vi "calibAnalyzeImage.vi"(0 "Input cluster":T1, 11 "error in":errorcluster) -> (4 "Output cluster":T1, 6 "Image out":T5(plugin-control), 12 "bottom border":sgl, 13 "left border":sgl, 14 "right border":sgl, 15 "error out":errorcluster)   [LabVIEW 2020]
doc: "Analyze image with a neural network, filter results and return calculated distance"
uses:
  controls/StateMachineVariables.ctl
  <vilib>/vision/Avi.llb/IMAQ AVI2 Refnum.ctl
  <vilib>/userDefined/High Color/IMAQdx.ctl
  <vilib>/vision/Deep Learning.llb/IMAQ DL Model Refnum.ctl
  <vilib>/vision/Image Controls.llb/IMAQ Image.ctl
  <vilib>/vision/Deep Learning.llb/IMAQ DL Model Detect Objects Node Names.ctl
  <vilib>/vision/Deep Learning.llb/IMAQ DL Model Label.ctl
  <vilib>/vision/NI_Vision_Development_Module.lvlib
panel:
  in  "Minimum Score Threshold":sgl=0.3 min=0 max=1 step=0.1 format="%.3g"
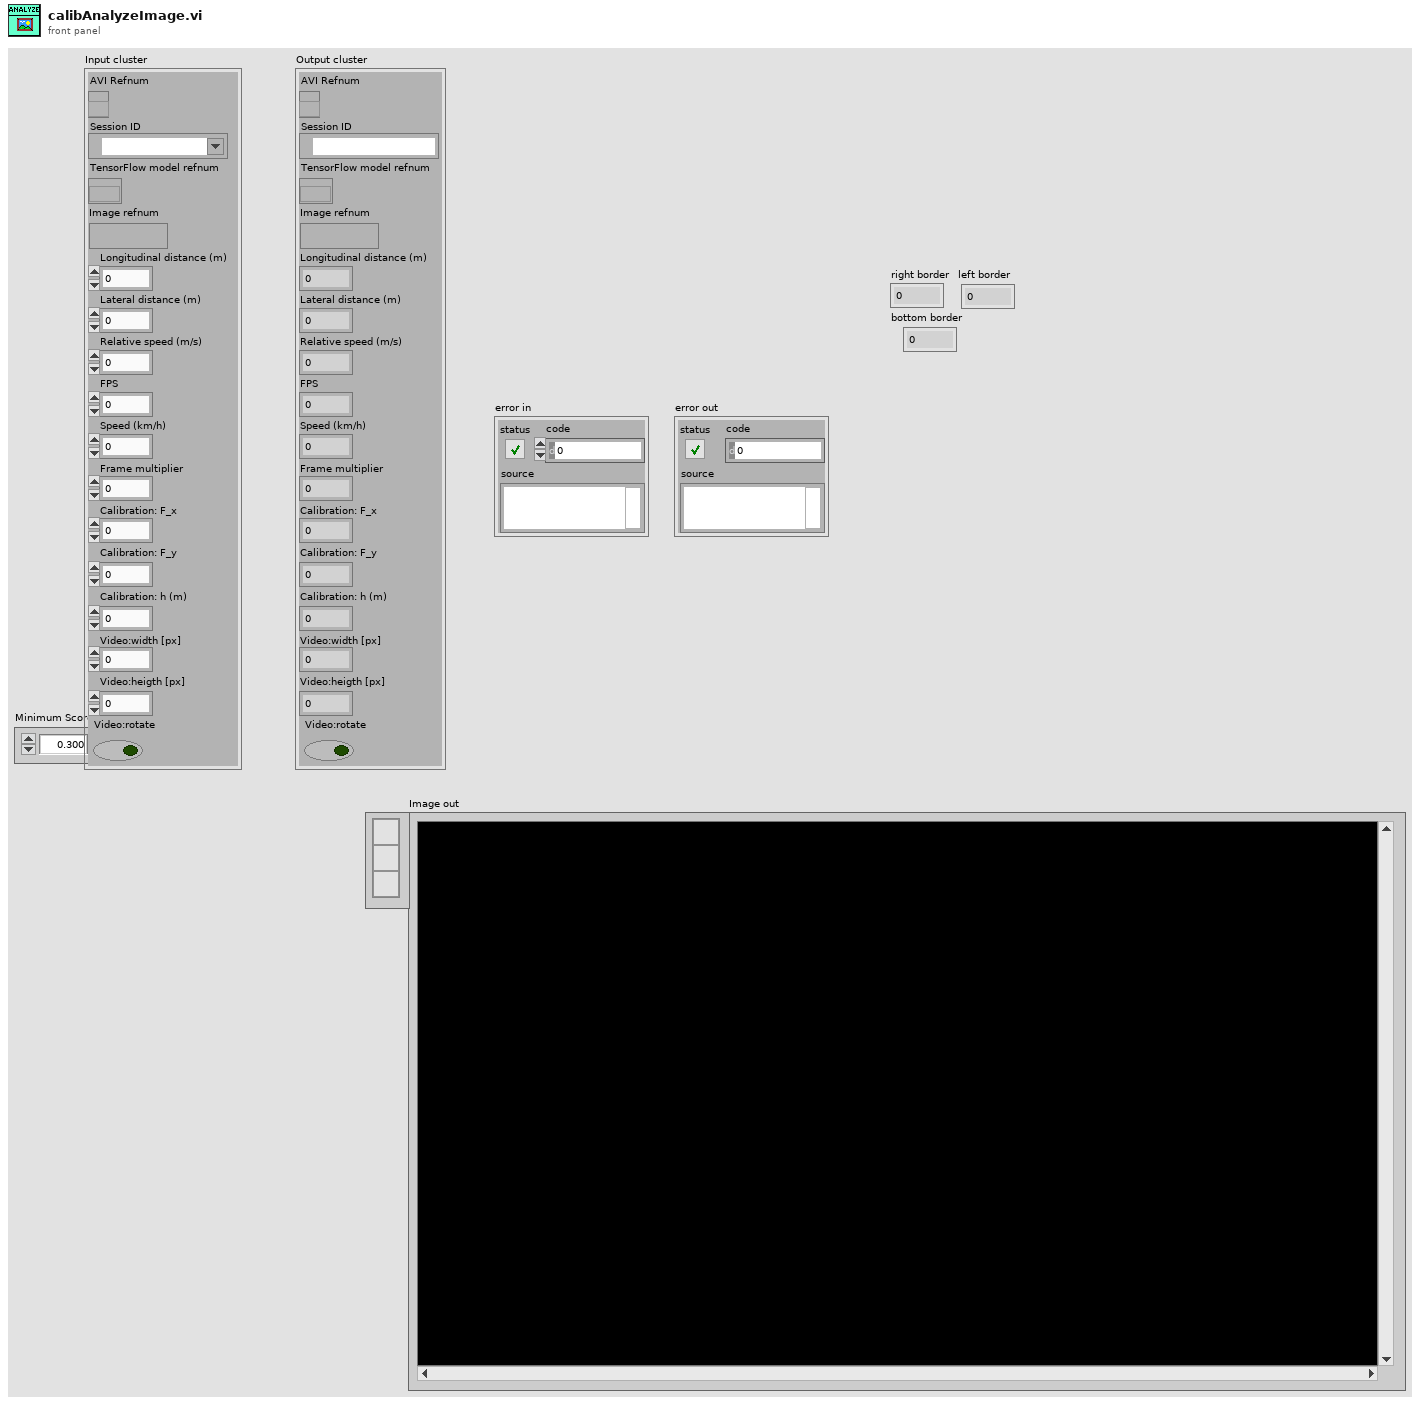
[diagram p1: front panel]
types:
  T1 = typedef "StateMachineVariables.ctl" = cluster{"AVI Refnum":T2, "Session ID":T3, "TensorFlow model refnum":T4, "Image refnum":T5, "Longitudinal distance (m)":dbl, "Lateral distance (m)":dbl, "Relative speed (m/s)":dbl, "FPS":dbl, "Speed (km/h)":dbl, "Frame multiplier":u32, "Calibration: F_x":dbl, "Calibration: F_y":dbl, "Calibration: h (m)":dbl, "Video:width [px]":i32, "Video:heigth [px]":i32, "Video:rotate":bool}
  T2 = typedef "IMAQ AVI2 Refnum.ctl" = refnum<k20>
  T3 = typedef "IMAQdx.ctl" = refnum<k21>
  T4 = typedef "IMAQ DL Model Refnum.ctl" = refnum<k20>
  T5 = typedef "IMAQ Image.ctl" = refnum<image>
  T6 = typedef "IMAQ DL Model Label.ctl" = cluster{"ID":u32, "Label":string}
  T7 = typedef "IMAQ DL Model Detect Objects Node Names.ctl" = cluster{"Number of Objects":string, "Labels":string, "Scores":string, "Bounding Boxes":string}
  T8 = typedef "IMAQ DL Model Output Data.ctl" = cluster{"Node Name":string, "Data":sgl[], "Dimensions":u64[]}
  T9 = typedef "IMAQ DL Model Objects.ctl" = cluster{"Label":string, "Score":sgl, "Bounding Box":cluster{"x":sgl, "y":sgl}[]}
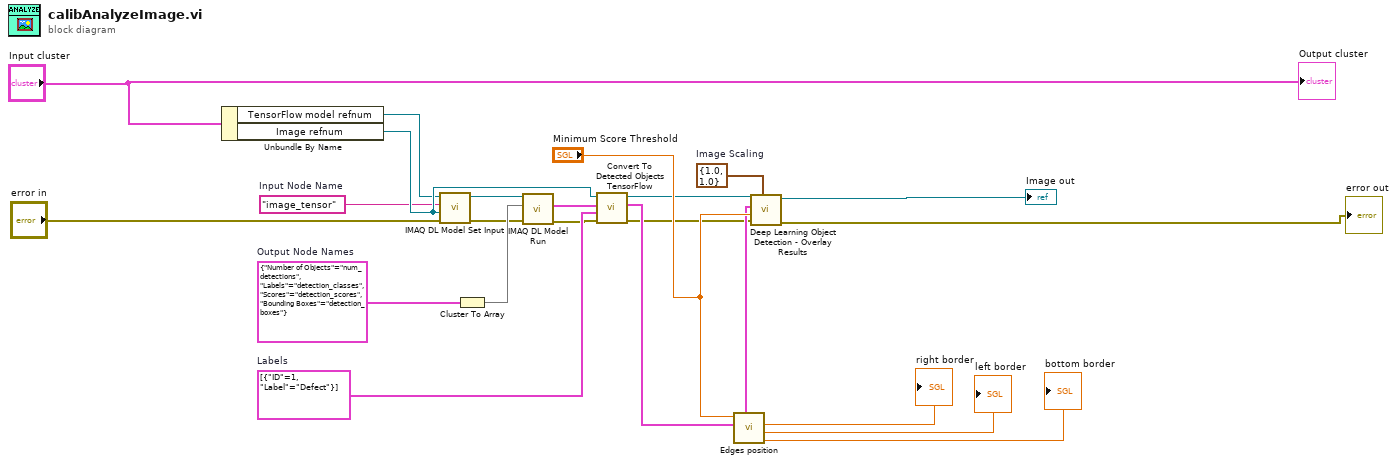
[diagram p0: block diagram]
diagram:
  w16 = T6[] [{"ID"=1, "Label"="Defect"}]  # Labels
  w14 = T7 {"Number of Objects"="num_detections", "Labels"="detection_classes", "Scores"="detection_scores", "Bounding Boxes"="detection_boxes"}  # Output Node Names
  w8 = "image_tensor"  # Input Node Name
  w7 = cluster{"X":dbl, "Y":dbl} {"X"=1.0, "Y"=1.0}  # Image Scaling
  n1 = Unbundle By Name("Input cluster") -> ("TensorFlow model refnum"=w20:T4, "Image refnum"=w22:T5)
  n2 = call-poly "IMAQ DL Model Set Input"("error in (no error)"="error in", "Image"=w22, "Input Node Name"=w8, "Model Refnum In"=w20) -> ("error out"=w10:errorcluster, "Model Refnum Out"=w9:T4)  [unwired: 5 in, 1 out]
  n3 = Cluster To Array(cluster=w14) -> (array=w15:string[])
  n4 = call "IMAQ DL Model Run"("error in (no error)"=w10, "Output Node Names"=w15, "Model Refnum In"=w9) -> ("error out"=w11:errorcluster, "Output Data Array"=w13:T8[])  [unwired: 6 in, 1 out]
  n5 = call "Convert To Detected Objects TensorFlow.vi"("error in (no error)"=w11, "Labels"=w16, "Output Data Array"=w13, "Image"=w22) -> ("error out"=w12:errorcluster, "Detected Objects"=w18:T9[], "Image (duplicate)"=w17:T5)  [unwired: 4 in, 1 out]
  n6 = call "Edges position.vi"("Detected Objects"=w18, "Minimum Score Threshold"="Minimum Score Threshold") -> ("bottom border"=→"bottom border":sgl, "left border"=→"left border":sgl, "right border"=→"right border":sgl, "nearest car object"=w19:T9[])  [unwired: 4 in, 2 out]
  n7 = call "Deep Learning Object Detection - Overlay Results.vi"("Image Scaling"=w7, "error in (no error)"=w12, "Minimum Score Threshold"="Minimum Score Threshold", "Detected Objects"=w19, "Image In"=w17) -> ("error out"=→"error out":errorcluster, "Image Out"=→"Image out":T5)  [unwired: 5 in]
  "Output cluster" <- "Input cluster"
